vi "analyzeImage.vi"(8 "error in":errorcluster, 9 "Height":dbl, 10 "Width":dbl, 11 "Input cluster":T1) -> (0 "error out":errorcluster, 1 "Cars found":i32, 2 "Car found":bool, 3 "Output cluster":T1, 4 "Distance":sgl(graph))   [LabVIEW 2020]
uses:
  controls/StateMachineVariables.ctl
  <vilib>/vision/Avi.llb/IMAQ AVI2 Refnum.ctl
  <vilib>/userDefined/High Color/IMAQdx.ctl
  <vilib>/vision/Deep Learning.llb/IMAQ DL Model Refnum.ctl
  <vilib>/vision/Image Controls.llb/IMAQ Image.ctl
  <vilib>/vision/Deep Learning.llb/IMAQ DL Model Detect Objects Node Names.ctl
  <vilib>/vision/Deep Learning.llb/IMAQ DL Model Label.ctl
  <vilib>/vision/NI_Vision_Development_Module.lvlib
panel:
  in  "Minimum Score Threshold":sgl=0.3 min=0 max=1 step=0.1 format="%.3g"
  out "Image out":T5(plugin-control)
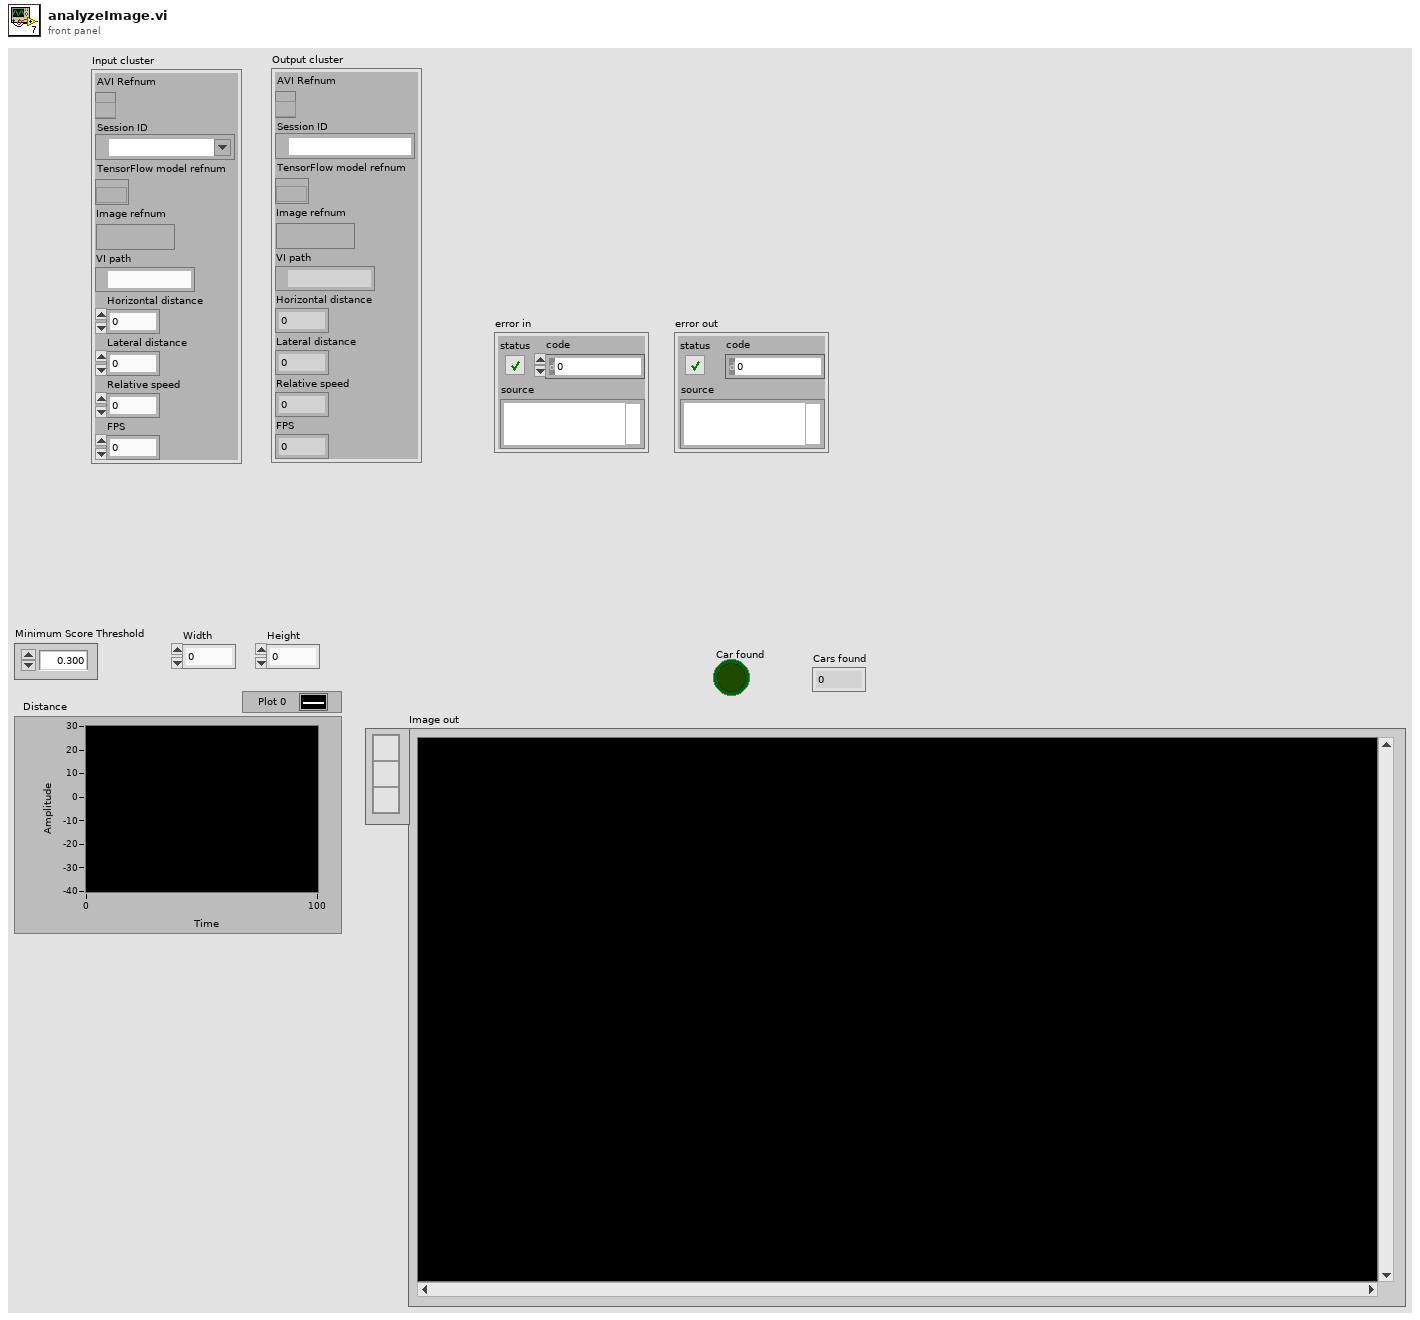
[diagram p1: front panel]
types:
  T1 = typedef "StateMachineVariables.ctl" = cluster{"AVI Refnum":T2, "Session ID":T3, "TensorFlow model refnum":T4, "Image refnum":T5, "VI path":path, "Horizontal distance":dbl, "Lateral distance":dbl, "Relative speed":dbl, "FPS":dbl}
  T2 = typedef "IMAQ AVI2 Refnum.ctl" = refnum<k20>
  T3 = typedef "IMAQdx.ctl" = refnum<k21>
  T4 = typedef "IMAQ DL Model Refnum.ctl" = refnum<k20>
  T5 = typedef "IMAQ Image.ctl" = refnum<image>
  T6 = typedef "IMAQ DL Model Label.ctl" = cluster{"ID":u32, "Label":string}
  T7 = typedef "IMAQ DL Model Detect Objects Node Names.ctl" = cluster{"Number of Objects":string, "Labels":string, "Scores":string, "Bounding Boxes":string}
  T8 = typedef "IMAQ DL Model Output Data.ctl" = cluster{"Node Name":string, "Data":sgl[], "Dimensions":u64[]}
  T9 = typedef "IMAQ DL Model Objects.ctl" = cluster{"Label":string, "Score":sgl, "Bounding Box":cluster{"x":sgl, "y":sgl}[]}
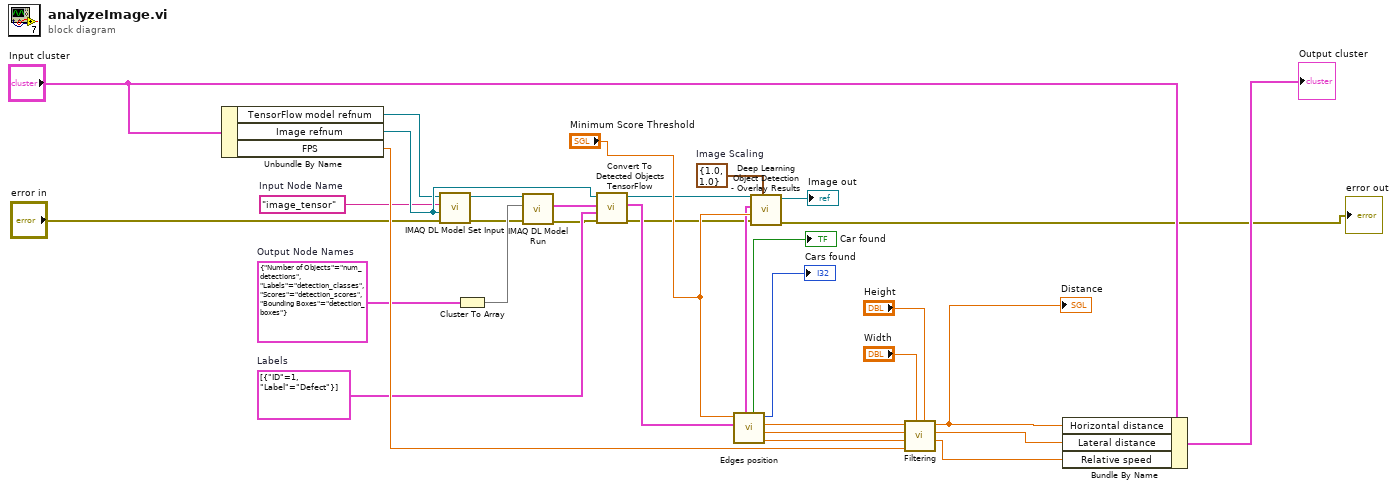
[diagram p0: block diagram]
diagram:
  w14 = T6[] [{"ID"=1, "Label"="Defect"}]  # Labels
  w12 = T7 {"Number of Objects"="num_detections", "Labels"="detection_classes", "Scores"="detection_scores", "Bounding Boxes"="detection_boxes"}  # Output Node Names
  w6 = "image_tensor"  # Input Node Name
  w5 = cluster{"X":dbl, "Y":dbl} {"X"=1.0, "Y"=1.0}  # Image Scaling
  n1 = Unbundle By Name("Input cluster") -> ("TensorFlow model refnum"=w23:T4, "Image refnum"=w28:T5, "FPS"=w31:dbl)
  n2 = call-poly "IMAQ DL Model Set Input"("error in (no error)"="error in", "Image"=w28, "Input Node Name"=w6, "Model Refnum In"=w23) -> ("error out"=w8:errorcluster, "Model Refnum Out"=w7:T4)  [unwired: 5 in, 1 out]
  n3 = Cluster To Array(cluster=w12) -> (array=w13:string[])
  n4 = call "IMAQ DL Model Run"("error in (no error)"=w8, "Output Node Names"=w13, "Model Refnum In"=w7) -> ("error out"=w9:errorcluster, "Output Data Array"=w11:T8[])  [unwired: 6 in, 1 out]
  n5 = call "Convert To Detected Objects TensorFlow.vi"("error in (no error)"=w9, "Labels"=w14, "Output Data Array"=w11, "Image"=w28) -> ("error out"=w10:errorcluster, "Detected Objects"=w18:T9[], "Image (duplicate)"=w15:T5)  [unwired: 4 in, 1 out]
  n6 = call "Edges position.vi"("Detected Objects"=w18, "Minimum Score Threshold"="Minimum Score Threshold") -> ("bottom border"=w22:sgl, "left border"=w21:sgl, "right border"=w20:sgl, "Cars found"=→"Cars found":i32, "Car found"=→"Car found":bool, "nearest car object"=w19:T9[])  [unwired: 4 in]
  n7 = call "Deep Learning Object Detection - Overlay Results.vi"("Image Scaling"=w5, "error in (no error)"=w10, "Minimum Score Threshold"="Minimum Score Threshold", "Detected Objects"=w19, "Image In"=w15) -> ("error out"=→"error out":errorcluster, "Image Out"=→"Image out":T5)  [unwired: 5 in]
  n8 = call "Filtering.vi"("Right border"=w20, "Left border"=w21, "Bottom border"=w22, "fps"=w31, "width"="Width", "height"="Height") -> ("distance"=w25:sgl, "lateral distance"=w26:sgl, "relative speed"=w27:sgl)  [unwired: 2 in]
  "Distance" <- w25
  n9 = Bundle By Name(cluster="Input cluster", "Horizontal distance"=w25, "Lateral distance"=w26, "Relative speed"=w27) -> (→"Output cluster":T1)
